vi "UHR-Fleezers Control (host) - 12.6.1.vi"() -> ()   [LabVIEW 2012] (continued)
            n2034 = Bundle("Left"=w2971, "Top"=w2970, "Width"=w2969, "Height"=w2968) -> (w2959:T33)  [unwired: 1 in]
            n2035 = Bundle("Left"=w2967, "Top"=w2966, "Width"=w2965, "Height"=w2964) -> (w2958:T33)  [unwired: 1 in]
            n2036 = Bundle("Left"=w2963, "Top"=w2962, "Width"=w2961, "Height"=w2960) -> (w2957:T33)  [unwired: 1 in]
            n2037 = Build Cluster Array(w2942, w2959, w2958, w2957) -> (w2956:T34)
            n2038 = for {
              tunnel: w2978 -> [w2989]
              tunnel: w2956 -> [w2990] mode=indexing
              shift-right: [w2987] -> w2954
              shift-left: TRUE -> [w2988]
              shift-right: [w2986] -> w2952
              shift-left: _ -> [w2982]
              shift-right: [w2985] -> w2951
              shift-left: _ -> [w2981]
              shift-right: [w2984] -> w2950
              shift-left: _ -> [w2980]
              shift-right: [w2983] -> w2949
              shift-left: _ -> [w2979]
              n2039 = case shown="True" w2988 {
                selector: w2988 -> [w2995 _]
                tunnel: w2990 -> [_ w3004]
                tunnel: w2989 -> [_ w3002]
                tunnel: [w2995 w3000] -> w2987
                tunnel: [w2994 w2999] -> w2986
                tunnel: [w2993 w2998] -> w2985
                tunnel: [w2992 w2997] -> w2984
                tunnel: [w2991 w2996] -> w2983
                tunnel: w2982 -> [w2994 _]
                tunnel: w2981 -> [w2993 _]
                tunnel: w2980 -> [w2992 _]
                tunnel: w2979 -> [w2991 _]
                frame False {
                }
                frame True {
                  n2040 = Unbundle(w3004) -> (w3003:T33)
                  n2041 = call "isclickinwindow.vi"("Image Param"=w3003, "Point32"=w3002) -> ("4 Y"=w2996:i32, "3 Height"=w2997:i32, "2 X"=w2998:i32, "1 Width"=w2999:i32, "In image?"=w3001:bool)  [unwired: 1 in]
                  n2042 = Not(x=w3001) -> (.not. x?=w3000:bool)
                }
              }
            }
            n2043 = Not(x=w2954) -> (.not. x?=w2953:bool)
            n2044 = case shown="True" w2953 {
              tunnel: w2951 -> [_ w3018]
              tunnel: w2949 -> [_ w3017]
              tunnel: w2952 -> [_ w3016]
              tunnel: w2950 -> [_ w3015]
              frame False {
              }
              frame True {
                w3005 = FALSE ("Get Point")
                n2045 = local read "Scan lines (y)"() -> (w3020:u64)
                n2046 = disable-structure shown="Disabled" {
                  frame Disabled {
                  }
                  frame Enabled {
                  }
                }
                n2047 = local read "Actual MCL Inc (V)"() -> (w3014:dbl)
                n2048 = local read "Scan steps (MCL)"() -> (w3019:u64)
                n2049 = Divide "Y Pix/step"(x=w3015, y=w3020) -> (x/y=w3027:dbl)
                n2050 = Divide "Y V/pix"(x=w3014, y=w3027) -> (x/y=w3026:dbl)
                n2051 = Divide "Y half step offset"(x=w3014, y=2.0) -> (x/y=w3028:dbl)
                n2052 = Divide "X pix/step"(x=w3016, y=w3019) -> (x/y=w3025:dbl)
                n2053 = Negate(x=w3028) -> (-x=w3029:dbl)
                n2054 = local read "Initial Y"() -> (w3035:dbl)
                n2055 = Multiply(x=w3017, y=w3026) -> (x*y=w3036:dbl)
                n2056 = Divide "X half step offset"(x=w3014, y=2.0) -> (x/y=w3022:dbl)
                n2057 = Divide "X V/pix"(x=w3014, y=w3025) -> (x/y=w3024:dbl)
                n2058 = Multiply(x=w3014, y=w3019) -> (x*y=w3031:dbl)
                n2059 = Compound Arithmetic op=ADD(w3029, w3036, w3035) -> (w3006:dbl)
                "Pointer Y (V)" <- w3006
                n2060 = Multiply(x=w3024, y=w3018) -> (x*y=w3033:dbl)
                n2061 = Negate(x=w3022) -> (-x=w3021:dbl)
                n2062 = local read "Initial X"() -> (w3034:dbl)
                n2063 = Negate(x=w3033) -> (-x=w3032:dbl)
                n2064 = Compound Arithmetic op=ADD(w3021, w3031, w3034, w3032) -> (w3007:dbl)
                "Pointer X (V)" <- w3007
                n2065 = case shown="True" "Set High F Confocal Spot (X-Y)" {
                  tunnel: w3007 -> [_ w3037]
                  tunnel: w3006 -> [_ w3038]
                  frame False {
                  }
                  frame True {
                    "Confocal Y 2 (V)" <- w3038
                    "Confocal X 2 (V)" <- w3037
                  }
                }
                n2066 = Or(x="Set X Only", y="Set Confocal Spot (X-Y)") -> (x .or. y?=w3010:bool)
                n2067 = Or(x="Set Confocal Spot (X-Y)", y="Set Y Only") -> (x .or. y?=w3009:bool)
                n2068 = case shown="True" w3010 {
                  tunnel: w3007 -> [_ w3039]
                  frame False {
                  }
                  frame True {
                    n2069 = property on="AO2" class="Slide (strict)"("Val(Sgnl)"=w3039) -> ()  [unwired: 2 in, 2 out]
                    "Confocal X 1 (V)" <- w3039
                  }
                }
                n2070 = case shown="True" w3009 {
                  tunnel: w3006 -> [_ w3040]
                  frame False {
                  }
                  frame True {
                    n2071 = property on="AO1" class="Slide (strict)"("Val(Sgnl)"=w3040) -> ()  [unwired: 2 in, 2 out]
                    "Confocal Y 1 (V)" <- w3040
                  }
                }
                n2072 = local write "Set High F Confocal Spot (X-Y)"(w3005) -> ()
                n2073 = local write "Set Confocal Spot (X-Y)"(w3005) -> ()
                n2074 = local write "Set X Only"(w3005) -> ()
                n2075 = local write "Set Y Only"(w3005) -> ()
              }
            }
          }
          frame 3 {
            n2076 = local read "BD 2 Frequency 1 (MHz)"() -> (w3041:dbl)
            n2077 = local read "BD 1 Frequency 1 (MHz)"() -> (w3042:dbl)
            n2078 = local write "Manipulating Trap"(TRUE ("Manipulating Trap")) -> ()
            n2079 = local write "Coords"(T7 {"Horizontal"=0, "Vertical"=0} ("Coords")) -> ()
            n2080 = while {
              tunnel: w3047 -> [w3052]
              tunnel: w3045 -> [w3051]
              tunnel: w3043 -> [w3050]
              tunnel: w3042 -> [w3049]
              tunnel: w3041 -> [w3048]
              stop <- w3053 stop-if-true
              n2081 = event shown="[0] \"Pane\": Mouse Move" {
                selector: _ -> [_ _]
                dyn-events: _ -> [_ _]
                timeout: _ -> [_ _]
                tunnel: ["Force Manip Abort" w3117] -> w3053
                tunnel: w3052 -> [w3060 _]
                tunnel: w3051 -> [w3058 _]
                tunnel: w3050 -> [w3057 _]
                tunnel: w3049 -> [w3056 _]
                tunnel: w3048 -> [w3055 _]
                event Mouse Move {
                  n2082 = event-data() -> ("Time"=w3061:u32, "Coords"=w3062:T7)  [unwired: 3 out]
                  n2083 = Less?(x=w3061, y=w3060) -> (x < y?=w3059:bool)
                  n2084 = case "Makes sure old motion events prior to mouse click aren't used" shown="False" w3059 {
                    tunnel: w3062 -> [w3104 _]
                    tunnel: w3058 -> [w3105 _]
                    tunnel: w3057 -> [w3082 _]
                    tunnel: w3056 -> [w3078 _]
                    tunnel: w3055 -> [w3077 _]
                    frame False {
                      n2085 = Subtract(x=w3104, y=w3105) -> (x-y=w3103:T7)
                      "Coords" <- w3103
                      n2086 = local read "Y RF Frequency Limits (MHz)"() -> (w3063:T16)
                      n2087 = To Double Precision Float(number=w3103) -> (double precision float=w3102:cluster{"Horizontal":dbl, "Vertical":dbl})
                      n2088 = Multiply(x=cluster{"Horizontal":dbl, "Vertical":dbl} {"Horizontal"=-1.0, "Vertical"=1.0}, y="Manipulation Scaling") -> (x*y=w3098:cluster{"Horizontal":dbl, "Vertical":dbl})
                      n2089 = local read "X RF Frequency Limits (MHz)"() -> (w3064:T16)
                      n2090 = Multiply(x=w3102, y=w3098) -> (x*y=w3100:cluster{"Horizontal":dbl, "Vertical":dbl})
                      n2091 = Unbundle By Name(w3100) -> ("Horizontal"=w3095:dbl, "Vertical"=w3099:dbl)
                      n2092 = Unbundle By Name(w3063) -> ("Maximum"=w3066:dbl, "Minimum"=w3065:dbl)
                      n2093 = Boolean To (0,1)(Boolean="Manip. X?") -> (0, 1=w3093:i16)
                      n2094 = Boolean To (0,1)(Boolean="Manip. Y?") -> (0, 1=w3090:i16)
                      n2095 = local read "BD 1 Frequency 2 (MHz)"() -> (w3080:dbl)
                      n2096 = Multiply(x=w3099, y=w3090) -> (x*y=w3092:dbl)
                      n2097 = Multiply(x=w3093, y=w3095) -> (x*y=w3096:dbl)
                      n2098 = local read "BD 2 Frequency 2 (MHz)"() -> (w3079:dbl)
                      n2099 = Unbundle By Name(w3064) -> ("Maximum"=w3068:dbl, "Minimum"=w3067:dbl)
                      n2100 = Add(x=w3077, y=w3092) -> (x+y=w3070:dbl)
                      n2101 = Add(x=w3078, y=w3096) -> (x+y=w3072:dbl)
                      n2102 = In Range and Coerce(upper limit=w3068, x=w3072, lower limit=w3067) -> (coerced(x)=w3071:dbl)  [unwired: 1 out]
                      n2103 = In Range and Coerce(upper limit=w3066, x=w3070, lower limit=w3065) -> (coerced(x)=w3069:dbl)  [unwired: 1 out]
                      n2104 = Subtract(x=w3071, y=w3080) -> (x-y=w3089:dbl)
                      n2105 = Subtract(x=w3069, y=w3079) -> (x-y=w3088:dbl)
                      n2106 = Square(x=w3089) -> (x^2=w3087:dbl)
                      n2107 = Square(x=w3088) -> (x^2=w3086:dbl)
                      n2108 = Add(x=w3087, y=w3086) -> (x+y=w3085:dbl)
                      n2109 = Square Root(x=w3085) -> (sqrt(x)=w3081:dbl)
                      n2110 = In Range and Coerce(upper limit="Limit Max (MHz)", x=w3081, lower limit="Limit Min (MHz)") -> (In Range?=w3074:bool)  [unwired: 1 out]
                      n2111 = Not(x="Limits Enable") -> (.not. x?=w3073:bool)
                      n2112 = Or(x=w3074, y=w3073) -> (x .or. y?=w3075:bool)
                      n2113 = case shown="True" w3075 {
                        tunnel: w3082 -> [_ w3115]
                        tunnel: w3081 -> [_ w3106]
                        tunnel: w3071 -> [_ w3113]
                        tunnel: w3080 -> [_ w3112]
                        tunnel: w3069 -> [_ w3111]
                        tunnel: w3079 -> [_ w3110]
                        tunnel: w3064 -> [_ w3108]
                        tunnel: w3063 -> [_ w3107]
                        frame False {
                        }
                        frame True {
                          n2114 = local read "BD 1 Frequency 3 (MHz)"() -> (w3114:dbl)
                          n2115 = local read "BD 2 Frequency 3 (MHz)"() -> (w3109:dbl)
                          n2116 = local write "Trap Delta (MHz)"(w3106) -> ()
                          n2117 = call "set RF board frequency - interlace.vi"("Board 2 Frequency Limits"=w3107, "Board 1 Frequency Limits"=w3108, "FPGA VI Reference In"=w3115, "Board 2 Frequency 3 (MHz)"=w3109, "Board 1 Frequency 3 (MHz)"=w3114, "Board 2 Frequency 2 (MHz)"=w3110, "Board 2 Frequency 1 (MHz)"=w3111, "Board 1 Frequency 2 (MHz)"=w3112, "Board 1 Frequency 1  (MHz)"=w3113) -> ()  [unwired: 1 in, 2 out]
                          n2118 = local write "BD 2 Frequency 1 (MHz)"(w3111) -> ()
                          n2119 = local write "BD 1 Frequency 1 (MHz)"(w3113) -> ()
                        }
                      }
                    }
                    frame True {
                    }
                  }
                }
                event Mouse Up {
                  n2120 = event-data() -> ("Button"=w3116:u16)  [unwired: 8 out]
                  n2121 = case shown="3" w3116 {
                    tunnel: [FALSE TRUE] -> w3117
                    frame 0, Default {
                    }
                    frame 3 {
                      n2122 = local read "Trap Delta (MHz)"() -> (w3119:dbl)
                      n2123 = property on="Initial delta (MHz)" class="DigNum (strict)"("Val(Sgnl)"=w3119) -> ()  [unwired: 2 in, 2 out]
                      n2124 = local write "Manipulating Trap"(FALSE ("Manipulating Trap")) -> ()
                    }
                  }
                }
              }
            }
          }
        }
      }
      event Mouse Move {
        n2125 = event-data() -> ()  [unwired: 6 out]
      }
    }
    n2126 = local read "Stop All"() -> (w2935:bool)
    n2127 = node-c288() -> ()  [unwired: 2 out]
  }
  n2128 = timed-loop "Main data acquisition loop (get data, process data for display, and save data to disk)" {
    tunnel: w16 -> [w3431]
    tunnel: w88 -> [w3430]
    tunnel: [w3460] -> w292
    tunnel: [w3455] -> w290
    timing: w200 -> [_]
    timing-out: [_] -> w199
    tunnel: w105 -> [w3284]
    stop <- "Stop All" stop-if-true
    w3201 = "Initialize"
    # "Fluorescence data into FIFO for external control vi's\n(e.g., fluorescence triggering) - Duncan Nall"
    n2129 = node-c288() -> ()  [unwired: 2 out]
    n2130 = First Call?() -> (First Call?: T/F=w3236:bool)
    n2131 = Or(x="Reset", y=w3236) -> (x .or. y?=w3237:bool)
    n2132 = local read "Flushing P1"() -> (w3156:bool)
    n2133 = case "Reset data stream (manual reset or at begining of some rastering and imaging)" shown="True" w3237 {
      tunnel: w3431 -> [w4502 w4510]
      tunnel: w3430 -> [w4501 w4509]
      tunnel: [w4502 w4504] -> w3426
      tunnel: [w4501 w4503] -> w3425
      frame False {
      }
      frame True {
        w4507 = TRUE ("AI to FIFO")
        n2134 = local write "Overflow (data lost)"(FALSE ("Overflow (data lost)")) -> ()
        n2135 = call "reset FPGA DMA.vi"("error in"=w4509, "FPGA VI Reference In"=w4510) -> ("error out"=w4505:errorcluster, "FPGA VI Reference Out"=w4506:T20)
        n2136 = xnode "Read/Write Control"("FPGA VI Reference In"=w4506, "error in"=w4505, "AI to FIFO"=w4507, "APD to FIFO"=w4507) -> ("FPGA VI Reference Out"=w4504:T20, "error out"=w4503:errorcluster)
      }
    }
    n2137 = case shown="True" w3156 {
      frame False {
      }
      frame True {
        n2138 = local read "Flush rate (uL/m) P1"() -> (w3490:dbl)
        n2139 = local read "HP1 Flush Time (s)"() -> (w3499:dbl)
        n2140 = local read "DMA Update Period (s)"() -> (w3493:dbl)
        n2141 = Divide(x=w3490, y=60.0) -> (x/y=w3491:dbl)
        n2142 = Divide(x=w3499, y=w3493) -> (x/y=w3488:dbl)
        n2143 = feedback #1(0) -> (w3497:i32)
        n2144 = Increment(x=w3497) -> (x+1=w3487:i32)
        n2145 = Greater?(x=w3487, y=w3488) -> (0:w3496:bool)
        n2146 = Compound Arithmetic op=MULTIPLY(w3493, w3487, w3491) -> (→"P1 Flush Volume (uL)":dbl)
        n2147 = Divide(x=w3487, y=w3488) -> (x/y=→"P1 Flushing Bar":dbl)
        n2148 = case shown="True" w3496 {
          tunnel: w3487 -> [w3500 _]
          tunnel: [w3500 0] -> w3495
          frame False {
          }
          frame True {
            w3501 = FALSE ("Flushing P1")
            n2149 = local write "Inject Pump 1"(w3501) -> ()
            n2150 = local write "Flushing P1"(w3501) -> ()
            n2151 = property on="Clear Volume P1" class="Bool (strict)"("Val(Sgnl)"=TRUE ("Value (Signaling)")) -> ()  [unwired: 2 in, 2 out]
          }
        }
        n2152 = feedback-in #1(w3495) -> ()
      }
    }
    n2153 = Or(x="Start AOD Scan", y="Trap Raster Scan") -> (x .or. y?=w3382:bool)
    n2154 = case "Start AOM raster scan" shown="True" w3382 {
      tunnel: w3426 -> [w4352 w4362]
      tunnel: w3425 -> [w4351 w4361]
      tunnel: [w4352 w4355] -> w3424
      tunnel: [w4351 w4354] -> w3423
      frame False {
      }
      frame True {
        n2155 = case shown="True" "Restart DMA? (AOD)" {
          tunnel: [w4400 w4402] -> w4356
          tunnel: [w4399 w4401] -> w4357
          tunnel: w4362 -> [w4400 w4404]
          tunnel: w4361 -> [w4399 w4403]
          frame False {
          }
          frame True {
            n2156 = local write "Overflow (data lost)"(FALSE ("Overflow (data lost)")) -> ()
            n2157 = call "reset FPGA DMA.vi"("error in"=w4403, "FPGA VI Reference In"=w4404) -> ("error out"=w4401:errorcluster, "FPGA VI Reference Out"=w4402:T20)
          }
        }
        n2158 = local write "Trap Raster Scan"(FALSE ("Trap Raster Scan")) -> ()
        n2159 = case shown="True" "Move MCL Also?" {
          tunnel: w4357 -> [w4365 w4394]
          tunnel: w4356 -> [w4366 w4395]
          tunnel: [w4364 w4398] -> w4355
          tunnel: [w4363 w4397] -> w4354
          frame False {
            w4367 = TRUE ("AI to FIFO")
            n2160 = xnode "Read/Write Control"("FPGA VI Reference In"=w4366, "error in"=w4365, "AI to FIFO"=w4367, "APD to FIFO"=w4367, "Start scan"=w4367) -> ("FPGA VI Reference Out"=w4364:T20, "error out"=w4363:errorcluster)
          }
          frame True {
            w4391 = FALSE ("1D or 2D Scan?")
            w4396 = TRUE ("AI to FIFO")
            # "Count for MCL loop"
            # "N total cycles"
            # "N steps"
            # "V_int"
            n2161 = local read "Scan Range (nm)"() -> (w4373:dbl)
            n2162 = local read "Number of F/B Scans (AOD)"() -> (w4390:u16)
            n2163 = Sign(1:w4373) -> (0:w4372:dbl)
            n2164 = Compound Arithmetic op=MULTIPLY(w4373, "MCL Step Position Ratio", "MCL/AOM Scale Tweak") -> (w4377:dbl)
            n2165 = Negate(x=w4372) -> (-x=w4369:dbl)
            n2166 = Multiply(x=w4369, y="MCL Step Increment (V_int)") -> (x*y=w4371:dbl)
            n2167 = Divide(x=w4377, y="MCL X Cal (nm/V)") -> (x/y=w4383:dbl)
            n2168 = Multiply(x=32767.0 ("y"), y=w4383) -> (x*y=w4389:dbl)
            n2169 = local read "Total Counts (ticks)"() -> (w4374:u16)
            n2170 = local read "Cycles/step (AOD)"() -> (w4385:u64)
            n2171 = local read "Scan steps (AOD)"() -> (w4386:u64)
            n2172 = Divide(x=w4389, y=10.0) -> (x/y=w4382:dbl)
            n2173 = Divide(x=w4382, y="MCL Step Increment (V_int)") -> (x/y=w4380:dbl)
            n2174 = Absolute Value(x=w4380) -> (abs(x)=w4368:dbl)
            n2175 = Compound Arithmetic op=MULTIPLY(w4386, w4385, w4374) -> (w4381:u64)
            n2176 = local write "wait to reset values"(w4396) -> ()
            n2177 = local write "MCL Scanning"(w4396) -> ()
            n2178 = Divide(x=w4381, y=w4368) -> (x/y=w4378:dbl)
            "MCL Count" <- w4378
            n2179 = xnode "Read/Write Control"("FPGA VI Reference In"=w4395, "error in"=w4394, "Scan steps (MCL)"=w4368, "Number of scans (MCL)"=w4390, "Cycles per step (MCL)"=u64 1, "Scan freq.  increment (MCL)"=w4371, "1D or 2D Scan?"=w4391, "MCL Scan Axis"=w4391, "Cont. Scan (MCL)"=w4391, "MCL count"=w4378) -> ("FPGA VI Reference Out"=w4393:T20, "error out"=w4392:errorcluster)
            n2180 = xnode "Read/Write Control"("FPGA VI Reference In"=w4393, "error in"=w4392, "AI to FIFO"=w4396, "APD to FIFO"=w4396, "Start scan"=w4396, "Start scan (MCL)"=w4396) -> ("FPGA VI Reference Out"=w4398:T20, "error out"=w4397:errorcluster)
          }
        }
        "Raster Scanning..." <- TRUE ("Scanning...")
      }
    }
    n2181 = local read "Flushing P3"() -> (w3157:bool)
    n2182 = case "Keep track of when Harvard Pump 3 is done flushing" shown="True" w3157 {
      frame False {
      }
      frame True {
        n2183 = local read "Flush rate (uL/m) P3"() -> (w3507:dbl)
        n2184 = local read "DMA Update Period (s)"() -> (w3509:dbl)
        n2185 = local read "HP3 Flush Time (s)"() -> (w3516:dbl)
        n2186 = Divide(x=w3507, y=60.0) -> (x/y=w3505:dbl)
        n2187 = feedback #2(0) -> (w3514:i32)
        n2188 = Increment(x=w3514) -> (x+1=w3508:i32)
        n2189 = Divide(x=w3516, y=w3509) -> (x/y=w3510:dbl)
        n2190 = Greater?(x=w3508, y=w3510) -> (0:w3513:bool)
        n2191 = Compound Arithmetic op=MULTIPLY(w3509, w3508, w3505) -> (→"P3 Flush Volume (uL)":dbl)
        n2192 = case shown="True" w3513 {
          tunnel: w3508 -> [w3517 _]
          tunnel: [w3517 0] -> w3512
          frame False {
          }
          frame True {
            w3518 = FALSE ("Flushing P3")
            n2193 = local write "Inject Pump 3"(w3518) -> ()
            n2194 = local write "Flushing P3"(w3518) -> ()
            n2195 = property on="Clear Volume P3" class="Bool (strict)"("Val(Sgnl)"=TRUE ("Value (Signaling)")) -> ()  [unwired: 2 in, 2 out]
          }
        }
        n2196 = feedback-in #2(w3512) -> ()
        n2197 = Divide(x=w3508, y=w3510) -> (x/y=→"P3 Flushing Bar":dbl)
      }
    }
    n2198 = And(x="Save scans", y=w3382) -> (x .and. y?=w3422:bool)
    n2199 = Compound Arithmetic op=OR("Start MCL Scan", "Confocal Image", "Confocal Linescan") -> (w3380:bool)
    n2200 = And(x="Save Data (MCL)", y=w3380) -> (x .and. y?=w3421:bool)
    n2201 = case "Start MCL raster scan" shown="True" w3380 {
      tunnel: w3424 -> [w3964 w3980]
      tunnel: w3423 -> [w3963 w3979]
      tunnel: [w3964 w3975] -> w3283
      tunnel: [w3963 w3974] -> w3282
      tunnel: [FALSE w3973] -> w3407
      tunnel: "Start MCL Scan" -> [_ w3968]
      tunnel: "Confocal Image" -> [_ w3967]
      tunnel: "Confocal Linescan" -> [_ _]
      frame False {
      }
      frame True {
        w3973 = TRUE
        n2202 = case shown="True" "Restart DMA? (MCL)" {
          tunnel: [w4025 w4027] -> w3978
          tunnel: [w4024 w4026] -> w3977
          tunnel: w3980 -> [w4025 w4030]
          tunnel: w3979 -> [w4024 w4029]
          frame False {
          }
          frame True {
            n2203 = call "reset FPGA DMA.vi"("error in"=w4029, "FPGA VI Reference In"=w4030) -> ("error out"=w4026:errorcluster, "FPGA VI Reference Out"=w4027:T20)
            n2204 = local write "Overflow (data lost)"(FALSE ("Overflow (data lost)")) -> ()
          }
        }
        n2205 = case shown="False" w3968 {
          selector: w3968 -> [_ w3984]
          tunnel: w3967 -> [w3983 _]
          tunnel: [w3983 w3984] -> w3966
          frame False {
            n2206 = property on="2D or 1D Scan" class="Bool (strict)"("Val(Sgnl)"=w3983) -> ()  [unwired: 2 in, 2 out]
            n2207 = property on="Confocal Image" class="Bool (strict)"("Value"=FALSE ("Start Confocal Map")) -> ()  [unwired: 2 in, 2 out]
          }
          frame True {
          }
        }
        n2208 = local write "MCL Scanning"(w3973) -> ()
        n2209 = local read "AO1"() -> (w3970:dbl)
        n2210 = local read "AO2"() -> (w3969:dbl)
        n2211 = case shown="True" "Center Scan" {
          tunnel: w3978 -> [w3991 w4023]
          tunnel: w3977 -> [w3990 w4022]
          tunnel: [w3989 w4021] -> w3975
          tunnel: [w3988 w4020] -> w3974
          tunnel: [w3986 w4007] -> w3972
          tunnel: [w3985 w4006] -> w3971
          tunnel: w3970 -> [w3986 w4012]
          tunnel: w3969 -> [w3985 w4015]
          tunnel: w3966 -> [_ _]
          frame False {
            w3987 = TRUE ("AI to FIFO")
            n2212 = xnode "Read/Write Control"("FPGA VI Reference In"=w3991, "error in"=w3990, "AI to FIFO"=w3987, "APD to FIFO"=w3987, "Start scan (MCL)"=w3987) -> ("FPGA VI Reference Out"=w3989:T20, "error out"=w3988:errorcluster)
          }
          frame True {
            w4019 = TRUE ("AI to FIFO")
            n2213 = local read "Scan steps (MCL)"() -> (w3998:u64)
            n2214 = local read "Scan lines (y)"() -> (w3994:u64)
            n2215 = local read "Fast Scan Dir"() -> (w4005:bool)
            n2216 = local read "Actual MCL Inc (V)"() -> (w3995:dbl)
            n2217 = Decrement(x=w3994) -> (x-1=w3993:u64)
            n2218 = Decrement(x=w3998) -> (x-1=w3997:u64)
            n2219 = Multiply(x=w3995, y=w3993) -> (x*y=w3992:dbl)
            n2220 = Divide(x=w3992, y=2.0) -> (x/y=w4002:dbl)
            n2221 = Multiply(x=w3995, y=w3997) -> (x*y=w3996:dbl)
            n2222 = Divide(x=w3996, y=2.0) -> (x/y=w4001:dbl)
            n2223 = Select(t=w4001, s=w4005, f=w4002) -> (s? t:f=w4000:dbl)
            n2224 = Select(t=w4002, s=w4005, f=w4001) -> (s? t:f=w4004:dbl)
            n2225 = Subtract(x=w4012, y=w4004) -> (x-y=w4003:dbl)
            n2226 = Subtract(x=w4015, y=w4000) -> (x-y=w3999:dbl)
            n2227 = local read "2D or 1D Scan"() -> (w4017:bool)
            n2228 = Not(x=w4005) -> (.not. x?=w4011:bool)
            n2229 = Not(x=w4017) -> (.not. x?=w4013:bool)
            n2230 = And(x=w4005, y=w4013) -> (x .and. y?=w4014:bool)
            n2231 = And(x=w4013, y=w4011) -> (x .and. y?=w4016:bool)
            n2232 = Select(t=w4015, s=w4016, f=w3999) -> (s? t:f=w4006:dbl)
            n2233 = Select(t=w4012, s=w4014, f=w4003) -> (s? t:f=w4007:dbl)
            n2234 = call "Volt to I16.vi"("Voltage In"=w4007) -> ("I16 Voltage Out"=w4010:i16)
            n2235 = call "Volt to I16.vi"("Voltage In"=w4006) -> ("I16 Voltage Out"=w4009:i16)
            n2236 = xnode "Read/Write Control"("FPGA VI Reference In"=w4023, "error in"=w4022, "AI to FIFO"=w4019, "APD to FIFO"=w4019, "Start scan (MCL)"=w4019, "AO1"=w4010, "AO2"=w4009) -> ("FPGA VI Reference Out"=w4021:T20, "error out"=w4020:errorcluster)
          }
        }
        "Initial Y" <- w3972
        "Initial X" <- w3971
        n2237 = local write "Tab Control 6"(T3."Imaging" ("Tab Control 6")) -> ()
        "wait to reset values" <- w3973
      }
    }
    n2238 = local read "APD Elements/DMA read"() -> (w3127:u32)
    n2239 = local read "Trap AI Elements/DMA read"() -> (w3345:u32)
    n2240 = xnode "Get APD Data"("FPGA VI Reference In"=w3283, "error in"=w3282, "Number of Elements"=w3127, "Timeout (ms)"=-1) -> ("Data"=w3314:u32[], "Elements Remaining"=→"APD FIFO Elements Remaining":u32)  [unwired: 2 out]
    n2241 = local read "Trap Pos Elements/DMA read"() -> (w3279:u32)
    n2242 = xnode "Invoke Method"("FPGA VI Reference In"=w3283, "error in"=w3282, "Number of Elements"=w3279, "Timeout (ms)"=-1) -> ("Data"=w3243:u16[], "Elements Remaining"=→"Trap Pos FIFO El Remaining":u32)  [unwired: 2 out]
    n2243 = xnode "Get Trap Data"("FPGA VI Reference In"=w3283, "error in"=w3282, "Number of Elements"=w3345, "Timeout (ms)"=-1 ("Timeout")) -> ("FPGA VI Reference Out"=w3178:T20, "error out"=w3177:errorcluster, "Data"=w3244:i16[], "Elements Remaining"=w3468:u32)
    "FIFO El. Rem." <- w3468
    n2244 = local read "DMA Update Period (s)"() -> (w3346:dbl)
    n2245 = local read "Trap AI FIFO Depth"() -> (w3470:u32)
    n2246 = local read "Number of APDs"() -> (w3146:u8)
    n2247 = Decimate 1D Array(w3243) -> (w3240:u16[], w3242:u16[], w3241:u16[])
    n2248 = feedback #3(0.0) -> (w3272:dbl)
    n2249 = Add(x=w3346, y=w3272) -> (x+y=w3444:dbl)
    n2250 = feedback-in #3(w3444) -> ()
    n2251 = To Time Stamp(1:w3272) -> (0:w3271:timestamp)
    n2252 = Subtract(x=w3470, y=w3345) -> (x-y=w3469:u32)
    n2253 = To Unsigned Long Integer(number=w3240) -> (unsigned 32bit integer=w3239:u32[])
    n2254 = Join Numbers(hi=w3242, lo=w3241) -> ((hi.lo)=w3238:u32[])
    n2255 = Divide(x=w3468, y=w3469) -> (x/y=w3467:dbl)
    "Buffer Status" <- w3467
    n2256 = case "Deinterlace APD signals" shown="3, Default" w3146 {
      tunnel: [w3480 w3486] -> w3126
      tunnel: w3314 -> [w3481 w3485]
      tunnel: [w3479 w3484] -> w3125
      tunnel: [w3478 w3482] -> w3123
      frame 3, Default {
        n2257 = Decimate 1D Array "APD signals"(w3481) -> (w3480:u32[], w3479:u32[], w3478:u32[])
      }
      frame 2 {
        n2258 = Decimate 1D Array "APD signals"(w3485) -> (w3486:u32[], w3484:u32[])
        n2259 = Multiply(x=w3484, y=u32 0) -> (x*y=w3482:u32[])
      }
    }
    n2260 = Join Numbers(hi=w3239, lo=w3238) -> ((hi.lo)=w3232:u64[])
    n2261 = call "IR AOM word to freq - vec.vi"("Frequency Word In (double vec)"=w3232) -> ("Frequency Out"=w3278:dbl[])
    n2262 = Equal?(x=w3467, y=1.0) -> (x = y?=w3465:bool)
    n2263 = case "Alert buffer overflow" shown="True" w3465 {
      frame False {
      }
      frame True {
        n2264 = call <vilib>:"Beep.vi"() -> ()  [unwired: 3 in, 9 out]
        "Overflow (data lost)" <- TRUE ("Overflow (data lost)")
      }
    }
    n2265 = Decimate 1D Array(w3278) -> (w3277:dbl[], w3276:dbl[])
    n2266 = Build Array(w3277, w3276) -> (w3275:dbl[][])
    n2267 = Bundle(w3126, w3125, w3123) -> (w3130:cluster{u32[], u32[], u32[]})  [unwired: 1 in]
    n2268 = Build Array(w3126, w3125, w3123) -> (w3404:u32[][])
    n2269 = for {
      tunnel: w3126 -> [w3476] mode=indexing
      n2270 = call "Smart Buffer (DBL) 1.vi"("new element [write]"=w3476, "mode"=T21."write") -> ()  [unwired: 4 in, 6 out]
    }
    n2271 = local read "APD Integration Time (s)"() -> (w3141:dbl)
    n2272 = To Double Precision Float(number=w3404) -> (double precision float=w3405:dbl[][])
    n2273 = feedback #4 "APD3"(w3123) -> (w3124:u32[])
    n2274 = feedback #5 "APD2"(w3125) -> (w3301:u32[])
    n2275 = feedback #6 "APD1"(w3126) -> (w3403:u32[])
    n2276 = Build Array (concatenate)(w3301, w3125) -> (w3300:u32[])
    n2277 = Build Array (concatenate)(w3124, w3123) -> (w3122:u32[])
    n2278 = Build Array (concatenate)(w3403, w3126) -> (w3400:u32[])
    n2279 = for {
      tunnel: w3125 -> [w3475] mode=indexing
      n2280 = call "Smart Buffer (DBL) 2.vi"("new element [write]"=w3475, "mode"=T21."write") -> ()  [unwired: 4 in, 6 out]
    }
    n2281 = Array Size(array=w3400) -> (size(s)=w3397:i32)
    n2282 = Array Size(array=w3126) -> (size(s)=w3399:i32)
    n2283 = Multiply(x=w3399, y="APD Ave N") -> (x*y=w3398:dbl)
    n2284 = Greater?(x=w3397, y=w3398) -> (0:w3401:bool)
    n2285 = Bundle("APD 1", "APD 2", "APD 3") -> (w3437:cluster{string, string, string})  [unwired: 1 out]
    n2286 = local read "Trap Sets"() -> (w3344:u32)
    n2287 = case shown="True" w3401 {
      tunnel: w3400 -> [w3779 w3788]
      tunnel: [w3779 w3786] -> w3351
      tunnel: w3398 -> [_ w3781]
      tunnel: w3397 -> [_ w3787]
      tunnel: w3300 -> [w3778 w3785]
      tunnel: [w3778 w3784] -> w3298
      tunnel: w3122 -> [w3777 w3783]
      tunnel: [w3777 w3780] -> w3142
      frame False {
      }
      frame True {
        n2288 = Subtract(x=w3787, y=w3781) -> (x-y=w3782:dbl)
        n2289 = Array Subset "APD3"(array=w3783, index=w3782, length=w3781) -> (w3780:u32[])
        n2290 = Array Subset "APD2"(array=w3785, index=w3782, length=w3781) -> (w3784:u32[])
        n2291 = Array Subset "APD1"(array=w3788, index=w3782, length=w3781) -> (w3786:u32[])
      }
    }
    n2292 = feedback-in #4(w3142) -> ()
    n2293 = feedback-in #5(w3298) -> ()
    n2294 = feedback-in #6(w3351) -> ()
    n2295 = Cluster To Array(cluster=w3437) -> (array=w3434:string[])
    n2296 = for "APD" {
      tunnel: w3405 -> [w4035] mode=indexing
      tunnel: w3141 -> [w4042]
      tunnel: [w4038] -> w3302 mode=indexing
      tunnel: "APD Disp. Scale" -> [w4039]
      tunnel: w3434 -> [w4037] mode=indexing
      tunnel: "APD Disp. Downsample" -> [w4033]
      tunnel: [w4036] -> w3433
      workers-P: _ -> [_]
      tunnel: w3271 -> [w4032]
      n2297 = call "integrate 1D array interval - double.vi"("Ave N"=w4033, "Array In"=w4035) -> ("Array Out"=w4034:dbl[])  [unwired: 1 out]
      n2298 = Multiply(x=w4042, y=w4033) -> (x*y=w4036:dbl)
      n2299 = Divide(x=w4034, y=w4039) -> (x/y=w4040:dbl[])
      n2300 = Bundle By Name("t0"=w4032, "Y"=w4040, "dt"=w4036) -> (w4041:waveform(dbl))  [unwired: 1 out]
      n2301 = Set Waveform Attribute(5:w4037, 6:"NI_ChannelName" ("name"), 7:w4041) -> (3:w4038:waveform(dbl))  [unwired: 1 in, 2 out]
    }
    "APD Display Period (s)" <- w3433
    n2302 = Reciprocal(x=w3433) -> (1/x=→"APD Display Freq. (Hz)":dbl)
    n2303 = case "Deinterlace trap data, average down PSD" shown="2" w3344 {
      tunnel: w3244 -> [w4060 w4125]
      tunnel: [w4057 w4122] -> w3337
      tunnel: [w4060 w4124] -> w3235
      tunnel: "Detector Type" -> [w4059 w4120]
      tunnel: [w4058 w4123] -> w3336
      tunnel: [w4056 w4121] -> w3442
      frame 1, Default {
        n2304 = Divide(x=w4060, y=3276.7) -> (x/y=w4061:dbl[])
        n2305 = Decimate 1D Array(w4061) -> (w4070:dbl[], w4069:dbl[], w4068:dbl[], w4067:dbl[], w4066:dbl[], w4065:dbl[], w4064:dbl[], w4063:dbl[])
        n2306 = case shown="\"IR-QPD + PSD + FB-QPD position\"" w4059 {
          tunnel: w4070 -> [w4094 w4119]
          tunnel: w4069 -> [w4093 w4118]
          tunnel: w4068 -> [w4078 w4096]
          tunnel: w4067 -> [w4079 w4106]
          tunnel: w4066 -> [w4092 w4117]
          tunnel: w4065 -> [w4091 w4116]
          tunnel: w4064 -> [w4075 w4097]
          tunnel: w4063 -> [w4074 w4095]
          tunnel: [w4073 w4103] -> w4058
          tunnel: [w4072 w4102] -> w4057
          tunnel: [w4071 w4101] -> w4056
          frame "IR-QPD + PSD + FB-QPD", Default {
            w4071 = 0  # Channel pattern
            n2307 = Divide(x=w4094, y=w4079) -> (x/y=w4081:dbl[])
            n2308 = Divide(x=w4093, y=w4079) -> (x/y=w4080:dbl[])
            n2309 = Divide(x=w4092, y=w4075) -> (x/y=w4077:dbl[])
            n2310 = Divide(x=w4091, y=w4074) -> (x/y=w4076:dbl[])
            n2311 = Build Array(w4081, w4080, w4079, w4078, w4077, w4076, w4075, w4074) -> (w4072:dbl[][])
            n2312 = Bundle("T1 Y", "T1 X", "T1 Sum", "FB Sum", "PSD Y", "PSD X", "PSD Y Sum", "PSD X Sum") -> (w4090:T41)  [unwired: 1 out]
            n2313 = Cluster To Array(cluster=w4090) -> (array=w4073:string[])
          }
          frame "IR-QPD + PSD + FB-QPD position" {
            w4101 = 3  # Channel pattern
            n2314 = Negate(x=w4097) -> (-x=w4098:dbl[])
            n2315 = Divide(x=w4119, y=w4106) -> (x/y=w4108:dbl[])
            n2316 = Divide(x=w4118, y=w4106) -> (x/y=w4107:dbl[])
            n2317 = Divide(x=w4117, y=w4097) -> (x/y=w4105:dbl[])
            n2318 = Divide(x=w4116, y=w4098) -> (x/y=w4104:dbl[])
            n2319 = Build Array(w4108, w4107, w4106, w4095, w4096, w4105, w4104, w4097) -> (w4102:dbl[][])
            n2320 = Bundle("T1 Y", "T1 X", "T1 Sum", "FB X", "FB Sum", "PSD Y", "PSD X", "PSD Y Sum") -> (w4115:T41)  [unwired: 1 out]
            n2321 = Cluster To Array(cluster=w4115) -> (array=w4103:string[])
          }
        }
      }
      frame 2 {
        n2322 = case shown="\"IR-QPD + PSD + FB-QPD X position\"" w4120 {
          tunnel: w4125 -> [w4187 w4259 w4330]
          tunnel: [w4126 w4250 w4261] -> w4124
          tunnel: [w4153 w4241 w4308] -> w4123
          tunnel: [w4152 w4204 w4275] -> w4122
          tunnel: [w4146 w4239 w4306] -> w4121
          frame "IR-QPD + PSD + FB-QPD", Default {
            w4146 = 1  # Channel pattern
            # "time average x2 the 4th signal and the 4 psd signals (detection laser)"
            # "deinterlace 3 signals from qpd"
            n2323 = Decimate 1D Array(w4187) -> (w4186:i16[], w4185:i16[], w4151:i16[], w4184:i16[], w4174:i16[], w4172:i16[], w4171:i16[], w4169:i16[])
            n2324 = Decimate 1D Array(w4151) -> (w4150:i16[], w4149:i16[])
            n2325 = Decimate 1D Array(w4186) -> (w4183:i16[], w4155:i16[])
            n2326 = Decimate 1D Array(w4185) -> (w4182:i16[], w4180:i16[])
            n2327 = Decimate 1D Array(w4184) -> (w4181:i16[], w4179:i16[])
            n2328 = call "downsample 1D array - double.vi"("Ave N"=2.0, "Array In"=w4174) -> ("Array Out"=w4173:dbl[])  [unwired: 1 out]
            n2329 = call "downsample 1D array - double.vi"("Ave N"=2.0, "Array In"=w4172) -> ("Array Out"=w4154:dbl[])  [unwired: 1 out]
            n2330 = call "downsample 1D array - double.vi"("Ave N"=2.0, "Array In"=w4171) -> ("Array Out"=w4170:dbl[])  [unwired: 1 out]
            n2331 = call "downsample 1D array - double.vi"("Ave N"=2.0, "Array In"=w4169) -> ("Array Out"=w4168:dbl[])  [unwired: 1 out]
            n2332 = Interleave 1D Arrays(w4183, w4182, w4181, w4155, w4180, w4179, w4150, w4149, w4173, w4154, w4170, w4168) -> (w4167:dbl[])
            n2333 = Divide(x=w4167, y=3276.7) -> (x/y=w4166:dbl[])
            n2334 = Decimate 1D Array(w4166) -> (w4165:dbl[], w4164:dbl[], w4163:dbl[], w4162:dbl[], w4161:dbl[], w4160:dbl[], w4148:dbl[], w4147:dbl[], w4159:dbl[], w4158:dbl[], w4157:dbl[], w4156:dbl[])
            n2335 = Divide(x=w4165, y=w4163) -> (x/y=w4133:dbl[])
            n2336 = Divide(x=w4164, y=w4163) -> (x/y=w4132:dbl[])
            n2337 = Divide(x=w4162, y=w4160) -> (x/y=w4131:dbl[])
            n2338 = Divide(x=w4161, y=w4160) -> (x/y=w4130:dbl[])
            n2339 = Divide(x=w4159, y=w4157) -> (x/y=w4129:dbl[])
            n2340 = Divide(x=w4158, y=w4156) -> (x/y=w4128:dbl[])
            n2341 = Build Array(w4133, w4132, w4163, w4131, w4130, w4160, w4148, w4147, w4129, w4128, w4157, w4156) -> (w4152:dbl[][])
            n2342 = Bundle("T1 Y", "T1 X", "T1 Sum", "T2 Y", "T2 X", "T2 Sum", "T1 FB Sum", "T2 FB Sum", "PSD Y", "PSD X", "PSD Y Sum", "PSD X Sum") -> (w4134:T42)  [unwired: 1 out]
            n2343 = To Word Integer(number=w4167) -> (16bit integer=w4126:i16[])
            n2344 = Cluster To Array(cluster=w4134) -> (array=w4153:string[])
          }
          frame "IR-QPD + PSD + FB-QPD X position" {
            w4239 = 2  # Channel pattern
            # "time average x2 the 3 psd signals (detection laser)"
            # "deinterlace 3 signals from qpds"
            n2345 = Decimate 1D Array(w4259) -> (w4258:i16[], w4257:i16[], w4240:i16[], w4256:i16[], w4202:i16[], w4199:i16[], w4196:i16[], w4227:i16[])
            n2346 = Select(t=i16 -1, s="Flip X Sign", f=i16 1) -> (s? t:f=w4192:i16)
            n2347 = Multiply(x=w4257, y=w4192) -> (x*y=w4193:i16[])
            n2348 = Decimate 1D Array(w4240) -> (w4225:i16[], w4223:i16[])
            n2349 = Decimate 1D Array(w4258) -> (w4255:i16[], w4242:i16[])
            n2350 = Decimate 1D Array(w4193) -> (w4254:i16[], w4252:i16[])
            n2351 = Decimate 1D Array(w4256) -> (w4253:i16[], w4251:i16[])
            n2352 = Decimate 1D Array(w4227) -> (w4226:i16[], w4224:i16[])
            n2353 = call "downsample 1D array - I16.vi"("Ave N"=2.0, "Array In"=w4202) -> ("Array Out"=w4200:i16[])  [unwired: 1 in]
            n2354 = call "downsample 1D array - I16.vi"("Ave N"=2.0, "Array In"=w4196) -> ("Array Out"=w4194:i16[])  [unwired: 1 in]
            n2355 = call "downsample 1D array - I16.vi"("Ave N"=2.0, "Array In"=w4199) -> ("Array Out"=w4197:i16[])  [unwired: 1 in]
            n2356 = Interleave 1D Arrays(w4255, w4254, w4253, w4242, w4252, w4251, w4226, w4225, w4224, w4223, w4200, w4197, w4194) -> (w4250:i16[])
            n2357 = Divide(x=w4250, y=3276.7) -> (x/y=w4249:dbl[])
            n2358 = Decimate 1D Array(w4249) -> (w4248:dbl[], w4247:dbl[], w4246:dbl[], w4245:dbl[], w4244:dbl[], w4243:dbl[], w4215:dbl[], w4213:dbl[], w4212:dbl[], w4210:dbl[], w4209:dbl[], w4208:dbl[], w4205:dbl[])
            n2359 = Negate(x=w4205) -> (-x=w4203:dbl[])
            n2360 = Divide(x=w4209, y=w4205) -> (x/y=w4207:dbl[])
            n2361 = Divide(x=w4208, y=w4203) -> (x/y=w4206:dbl[])
            n2362 = Divide(x=w4248, y=w4246) -> (x/y=w4231:dbl[])
            n2363 = Divide(x=w4247, y=w4246) -> (x/y=w4230:dbl[])
            n2364 = Divide(x=w4245, y=w4243) -> (x/y=w4229:dbl[])
            n2365 = Divide(x=w4244, y=w4243) -> (x/y=w4228:dbl[])
            n2366 = Divide(x=w4215, y=w4213) -> (x/y=w4214:dbl[])
            n2367 = Divide(x=w4212, y=w4210) -> (x/y=w4211:dbl[])
            n2368 = Build Array(w4231, w4230, w4246, w4229, w4228, w4243, w4214, w4213, w4211, w4210, w4207, w4206, w4205) -> (w4204:dbl[][])
            n2369 = Bundle("T1 Y", "T1 X", "T1 Sum", "T2 Y", "T2 X", "T2 Sum", "T1 FB X", "T1 FB Sum", "T2 FB X", "T2 FB Sum", "PSD Y", "PSD X", "PSD Y Sum") -> (w4232:T43)  [unwired: 1 out]
            n2370 = Cluster To Array(cluster=w4232) -> (array=w4241:string[])
          }
          frame "IR-QPD + PSD + FB-QPD XY positions" {
            w4306 = 4  # Channel pattern
            # "time average x2 the 3 psd signals (detection laser)"
            # "deinterlace 3 signals from qpds"
            n2371 = Decimate 1D Array(w4330) -> (w4329:i16[], w4328:i16[], w4307:i16[], w4327:i16[], w4273:i16[], w4319:i16[], w4318:i16[], w4295:i16[])
            n2372 = Decimate 1D Array "Feedback Sum"(w4307) -> (w4291:i16[], w4289:i16[])
            n2373 = Decimate 1D Array "QPD Y"(w4329) -> (w4326:i16[], w4309:i16[])
            n2374 = Decimate 1D Array "QPD X"(w4328) -> (w4325:i16[], w4323:i16[])
            n2375 = Decimate 1D Array "Feedback Y"(w4273) -> (w4272:i16[], w4271:i16[])
            n2376 = Decimate 1D Array "QPD Sum"(w4327) -> (w4324:i16[], w4322:i16[])
            n2377 = Decimate 1D Array "Feedback X"(w4295) -> (w4292:i16[], w4290:i16[])
            n2378 = call "downsample 1D array - double.vi"("Ave N"=2.0, "Array In"=w4319) -> ("Array Out"=w4294:dbl[])  [unwired: 1 out]
            n2379 = call "downsample 1D array - double.vi"("Ave N"=2.0, "Array In"=w4318) -> ("Array Out"=w4293:dbl[])  [unwired: 1 out]
            n2380 = Interleave 1D Arrays(w4326, w4325, w4324, w4309, w4323, w4322, w4272, w4292, w4291, w4271, w4290, w4289, w4294, w4293) -> (w4317:dbl[])
            n2381 = Divide(x=w4317, y=3276.7) -> (x/y=w4316:dbl[])
            n2382 = Decimate 1D Array(w4316) -> (w4315:dbl[], w4314:dbl[], w4313:dbl[], w4312:dbl[], w4311:dbl[], w4310:dbl[], w4268:dbl[], w4282:dbl[], w4266:dbl[], w4267:dbl[], w4280:dbl[], w4264:dbl[], w4278:dbl[], w4276:dbl[])
            n2383 = Negate(x=w4276) -> (-x=w4274:dbl[])
            n2384 = Divide(x=w4278, y=w4274) -> (x/y=w4277:dbl[])
            n2385 = Divide(x=w4267, y=w4264) -> (x/y=w4263:dbl[])
            n2386 = Divide(x=w4268, y=w4266) -> (x/y=w4265:dbl[])
            n2387 = Divide(x=w4315, y=w4313) -> (x/y=w4299:dbl[])
            n2388 = Divide(x=w4314, y=w4313) -> (x/y=w4298:dbl[])
            n2389 = Divide(x=w4312, y=w4310) -> (x/y=w4297:dbl[])
            n2390 = Divide(x=w4311, y=w4310) -> (x/y=w4296:dbl[])
            n2391 = Divide(x=w4282, y=w4266) -> (x/y=w4281:dbl[])
            n2392 = Divide(x=w4280, y=w4264) -> (x/y=w4279:dbl[])
            n2393 = Build Array(w4299, w4298, w4313, w4297, w4296, w4310, w4265, w4281, w4266, w4263, w4279, w4264, w4277, w4276) -> (w4275:dbl[][])
            n2394 = Bundle("T1 Y", "T1 X", "T1 Sum", "T2 Y", "T2 X", "T2 Sum", "T1 FB Y", "T1 FB X", "T1 FB Sum", "T2 FB Y", "T2 FB X", "T2 FB Sum", "PSD X", "PSD Y Sum") -> (w4262:T44)  [unwired: 1 out]
            n2395 = To Word Integer(number=w4317) -> (16bit integer=w4261:i16[])
            n2396 = Cluster To Array(cluster=w4262) -> (array=w4308:string[])
          }
        }
      }
    }
    "AI labels" <- w3336
    n2397 = local read "APD Integration Time (s)"() -> (w3309:dbl)
    n2398 = Array Size(array=w3351) -> (size(s)=w3396:i32)
    n2399 = call <vilib>:"Std Deviation and Variance.vi"("X"=w3298) -> ("standard deviation"=w3297:dbl)  [unwired: 1 in, 2 out]
    n2400 = Add Array Elements(numeric array=w3298) -> (sum=w3299:u32)
    n2401 = Add Array Elements(numeric array=w3351) -> (sum=w3406:u32)
    n2402 = call <vilib>:"Std Deviation and Variance.vi"("X"=w3351) -> ("standard deviation"=w3350:dbl)  [unwired: 1 in, 2 out]
    n2403 = Divide(x=w3297, y=w3141) -> (x/y=w3294:dbl)
    "Rate sigma (Hz) 2" <- w3294
    n2404 = Multiply(x=w3141, y=w3396) -> (x*y=w3143:dbl)
    "Int. Time (s)" <- w3143
    n2405 = Divide(x=w3299, y=w3143) -> (x/y=w3295:dbl)
    "APD 2 Rate (Hz)" <- w3295
    n2406 = Multiply(x="APD Disp. Scale", y=w3302) -> (x*y=w3311:waveform(dbl)[])
    n2407 = Divide(x=w3406, y=w3143) -> (x/y=w3348:dbl)
    "APD 1 Rate (Hz)" <- w3348
    n2408 = Divide(x=w3350, y=w3141) -> (x/y=w3349:dbl)
    "Rate sigma (Hz)" <- w3349
    n2409 = Divide(x=w3294, y=w3295) -> (x/y=→"Sigma/Mean 2":dbl)
    n2410 = Multiply(x="APD Disp. Downsample", y=w3309) -> (x*y=w3307:dbl)
    n2411 = Divide(x=w3349, y=w3348) -> (x/y=→"Sigma/Mean":dbl)
    n2412 = Divide(x=w3311, y=w3307) -> (x/y=w3133:waveform(dbl)[])
    n2413 = Index Array(array=w3133, index=0) -> (element=w3291:waveform(dbl))
    n2414 = Index Array(array=w3133, index=1) -> (element=w3289:waveform(dbl))
    n2415 = Index Array(array=w3133, index=2) -> (element=w3135:waveform(dbl))
    n2416 = Subtract(x=w3291, y="APD 1 Offset") -> (x-y=w3287:waveform(dbl))
    n2417 = Subtract(x=w3289, y="APD 2 Offset") -> (x-y=w3286:waveform(dbl))
    n2418 = Subtract(x=w3135, y="APD 3 Offset") -> (x-y=w3132:waveform(dbl))
    n2419 = Add Array Elements(numeric array=w3142) -> (sum=w3145:u32)
    n2420 = call <vilib>:"Std Deviation and Variance.vi"("X"=w3142) -> ("standard deviation"=w3144:dbl)  [unwired: 1 in, 2 out]
    n2421 = Build Array(w3287, w3286, w3132) -> (→"APD Chart":waveform(dbl)[])
    n2422 = Divide(x=w3145, y=w3143) -> (x/y=w3139:dbl)
    "APD 3 Rate (Hz)" <- w3139
    n2423 = Divide(x=w3144, y=w3141) -> (x/y=w3140:dbl)
    "Rate sigma (Hz) 3" <- w3140
    n2424 = Divide(x=w3140, y=w3139) -> (x/y=→"Sigma/Mean 3":dbl)
    n2425 = local read "Data Period (s)"() -> (w3194:dbl)
    n2426 = local read "BD 1 Frequency 2 (MHz)"() -> (w3227:dbl)
    n2427 = local read "BD 1 Frequency 1 (MHz)"() -> (w3228:dbl)
    n2428 = Decimate 1D Array(w3235) -> (w3259:i16[], w3258:i16[], w3256:i16[], w3255:i16[])  [unwired: 9 out]
    n2429 = Multiply(x=w3194, y="Trap Pos. Disp. Downsample") -> (x*y=w3192:dbl)
    n2430 = Divide(x=w3259, y=w3258) -> (x/y=w3260:dbl[])
    n2431 = Divide(x=w3256, y=w3255) -> (x/y=w3257:dbl[])
    n2432 = local read "AOM X Cal (nm/MHz)"() -> (w3225:dbl)
    n2433 = Split 1D Array(array=w3260, index="N El. to Ave.") -> (second subarray=w3263:dbl[])  [unwired: 1 out]
    n2434 = Split 1D Array(array=w3257, index="N El. to Ave.") -> (second subarray=w3262:dbl[])  [unwired: 1 out]
    n2435 = Multiply(x=w3194, y="Trap Disp. Downsample") -> (x*y=w3273:dbl)
    "Display Period (s)" <- w3273
    n2436 = for "Trap AI" {
      tunnel: [w4055] -> w3438 mode=indexing
      tunnel: w3271 -> [w4046]
      tunnel: "Trap Disp. Downsample" -> [w4053]
      tunnel: w3337 -> [w4051] mode=indexing
      tunnel: w3194 -> [w4050]
      tunnel: w3336 -> [w4049] mode=indexing
      tunnel: [w4048] -> w3306 mode=indexing
      tunnel: w3273 -> [w4047]
      workers-P: _ -> [_]
      n2437 = Bundle By Name("Y"=w4051, "dt"=w4050) -> (w4052:waveform(dbl))  [unwired: 1 out]
      n2438 = Set Waveform Attribute(5:w4049, 6:"NI_ChannelName" ("name"), 7:w4052) -> (3:w4048:waveform(dbl))  [unwired: 1 in, 2 out]
      n2439 = call "downsample 1D array - double.vi"("Ave N"=w4053, "Array In"=w4051) -> ("Array Out"=w4054:dbl[])  [unwired: 1 out]
      n2440 = Bundle By Name(cluster=w4048, "t0"=w4046, "Y"=w4054, "dt"=w4047) -> (w4055:waveform(dbl))
    }
    n2441 = Bundle("BD 1 Frequency 1 (MHz)"=w3228, "BD 1 Frequency 2 (MHz)"=w3227) -> (w3229:T45)  [unwired: 1 out]
    n2442 = call-poly <vilib>:"Mean.vi"("X"=w3262) -> ("mean"=w3250:dbl)  [unwired: 1 out]
    n2443 = call-poly <vilib>:"Mean.vi"("X"=w3263) -> ("mean"=w3251:dbl)  [unwired: 1 out]
    n2444 = Reciprocal(x=w3273) -> (1/x=→"Trap Disp. Freq. (Hz)":dbl)
    n2445 = Cluster To Array(cluster=w3229) -> (array=w3226:dbl[])
    n2446 = local read "Trap X AI1 (DMA)"() -> (w3261:T13)
    n2447 = local read "Data points/scans (MCL)"() -> (w3416:dbl)
    n2448 = To Fixed-Point(number=w3250) -> (fixed-point=w3248:fxp<+/-,16,1>)  [unwired: 1 in]
    n2449 = To Fixed-Point(number=w3251) -> (fixed-point=w3249:fxp<+/-,16,1>)  [unwired: 1 in]
    n2450 = Bundle("Trap 1 Pos.", "Trap 2 Pos.") -> (w3270:cluster{string, string})  [unwired: 1 out]
    n2451 = Bundle By Name(cluster=w3261, "Set 1"=w3249, "Set 2"=w3248) -> (→"Trap X AI1 (DMA)":T13)
    n2452 = Cluster To Array(cluster=w3270) -> (array=w3267:string[])
    n2453 = Unbundle(w3130) -> (w3131:u32[])  [unwired: 2 out]
    n2454 = Select(t=-1.0, s="Negate Y Axis", f=1.0) -> (s? t:f=w3211:dbl)
    n2455 = for "Trap Position" {
      tunnel: w3275 -> [w3646] mode=indexing
      tunnel: "Trap Pos. Disp. Downsample" -> [w3645]
      tunnel: w3192 -> [w3643]
      tunnel: w3271 -> [w3642]
      tunnel: w3267 -> [w3640] mode=indexing
      tunnel: [w3639] -> w3181 mode=indexing
      tunnel: w3226 -> [w3637] mode=indexing
      tunnel: w3225 -> [w3635]
      tunnel: w3211 -> [w3634]
      n2456 = call "downsample 1D array - double.vi"("Ave N"=w3645, "Array In"=w3646) -> ("Array Out"=w3644:dbl[])  [unwired: 1 out]
      n2457 = Subtract(x=w3644, y=w3637) -> (x-y=w3638:dbl[])
      n2458 = Multiply(x=w3635, y=w3638) -> (x*y=w3636:dbl[])
      n2459 = Multiply(x=w3634, y=w3636) -> (x*y=w3633:dbl[])
      n2460 = Bundle By Name("Y"=w3633, "dt"=w3643, "t0"=w3642) -> (w3641:waveform(dbl))  [unwired: 1 out]
      n2461 = Set Waveform Attribute(5:w3640, 6:"NI_ChannelName" ("name"), 7:w3641) -> (3:w3639:waveform(dbl))  [unwired: 1 in, 2 out]
    }
    n2462 = To Double Precision Float(number=w3131) -> (double precision float=w3334:dbl[])
    n2463 = local read "Display Period (s)"() -> (w3323:dbl)
    n2464 = Increment(x=w3416) -> (x+1=w3417:dbl)
    n2465 = Index Array(array=w3181, index=0) -> (element=w3185:waveform(dbl))
    n2466 = Index Array(array=w3181, index=1) -> (element=w3180:waveform(dbl))
    n2467 = feedback #7(w3417) -> (w3420:dbl)
    n2468 = Select(t=0, s=w3407, f=w3420) -> (s? t:f=w3413:dbl)
    n2469 = Array Size(array=w3334) -> (size(s)=w3419:i32)
    n2470 = Build Array (concatenate)(w3302, w3438) -> (w3304:waveform(dbl)[])
    "All Signals" <- w3304
    n2471 = Add(x=w3419, y=w3413) -> (x+y=w3414:dbl)
    n2472 = Unbundle By Name(w3185) -> ("Y"=w3186:dbl[])
    n2473 = Divide(x="Bead Sep. Int. Time (s)", y=w3323) -> (x/y=w3221:dbl)
    n2474 = Add(x=w3186, y="FB Trap Pos Offset") -> (x+y=w3184:dbl[])
    "T1 x pos data" <- w3184
    n2475 = Greater?(x=w3414, y=w3416) -> (0:w3415:bool)
    n2476 = feedback #8(w3184) -> (w3223:dbl[])
    n2477 = Build Array (concatenate)(w3184, w3223) -> (w3222:dbl[])
    n2478 = Bundle By Name(cluster=w3185, "Y"=w3184) -> (w3183:waveform(dbl))
    n2479 = Select(t=w3413, s=w3415, f=w3414) -> (s? t:f=w3412:dbl)
    n2480 = feedback-in #7(w3412) -> ()
    n2481 = local read "MCL Scanning"() -> (w3410:bool)
    n2482 = Bundle(w3183, w3180) -> (w3179:cluster{waveform(dbl), waveform(dbl)})  [unwired: 1 out]
    n2483 = Split 1D Array(array=w3222, index=w3221) -> (first subarray=w3215:dbl[])  [unwired: 1 out]
    n2484 = feedback-in #8(w3215) -> ()
    n2485 = Not(x=w3415) -> (.not. x?=w3409:bool)
    n2486 = Cluster To Array(cluster=w3179) -> (array=w3155:waveform(dbl)[])
    "Trap Positions" <- w3155
    n2487 = call-poly <vilib>:"Mean.vi"("X"=w3215) -> ("mean"=w3214:dbl)  [unwired: 1 out]
    "Mean T1 Position (nm)" <- w3214
    n2488 = Subtract(x=w3215, y=w3214) -> (x-y=w3220:dbl[])
    n2489 = Square(x=w3220) -> (x^2=w3219:dbl[])
    n2490 = And(x=w3409, y=w3410) -> (x .and. y?=w3411:bool)
    n2491 = call-poly <vilib>:"Mean.vi"("X"=w3219) -> ("mean"=w3218:dbl)  [unwired: 1 out]
    n2492 = Square Root(x=w3218) -> (sqrt(x)=w3217:dbl)
    n2493 = Or(x=w3411, y=w3407) -> (x .or. y?=w3408:bool)
    n2494 = Equal?(x="Tab Control 6", y=T35."High Res Display") -> (x = y?=w3340:bool)
    n2495 = Multiply(x=10.0, y=w3217) -> (x*y=→"Trap 1 Position RMS (A)":dbl)
    n2496 = case "For displaying the high resolution display (no downsampling)" shown="True" w3340 {
      tunnel: w3306 -> [_ w3666]
      frame False {
      }
      frame True {
        n2497 = Index Array(array=w3666, index="High Res. Display") -> (element=w3667:waveform(dbl))
        n2498 = call <vilib>:"Std Deviation and Variance.vi"("X"=w3667) -> ("mean"=w3674:dbl, "standard deviation"=w3679:dbl)  [unwired: 1 in, 1 out]
        "Mean Intensity" <- w3674
        "Sigma" <- w3679
        n2499 = Subtract(x=w3667, y=w3674) -> (x-y=w3673:waveform(dbl))
        n2500 = Select(t=w3673, s="Subtract mean", f=w3667) -> (s? t:f=→"1 Channel":waveform(dbl))
        n2501 = Divide(x=w3679, y=w3674) -> (x/y=→"Sigma/Mean":dbl)
        n2502 = feedback #9(1) -> (w3668:i32)
        n2503 = Greater Or Equal?(x=w3668, y="Slow mean N ave.") -> (x >= y?=w3681:bool)
        n2504 = Increment(x=w3668) -> (x+1=w3683:i32)
        n2505 = Select(t=1, s=w3681, f=w3683) -> (s? t:f=w3670:i32)
        n2506 = feedback-in #9(w3670) -> ()
        n2507 = feedback #10() -> (w3671:waveform(dbl))  [unwired: 1 out]
        n2508 = case shown="Default" w3668 {
          tunnel: [w3686 w3689] -> w3672
          tunnel: w3671 -> [w3688 _]
          tunnel: w3667 -> [w3687 w3689]
          frame Default {
            n2509 = call-poly <vilib>:"Append Waveforms.vi"("waveform B"=w3687, "waveform A"=w3688) -> ("waveform out"=w3686:waveform(dbl))  [unwired: 1 in, 8 out]
          }
          frame 1 {
          }
        }
        n2510 = feedback-in #10(w3672) -> ()
        n2511 = case shown="True" w3681 {
          tunnel: w3672 -> [_ w3685]
          frame False {
          }
          frame True {
            n2512 = call-poly <vilib>:"Mean.vi"("X"=w3685) -> ("mean"=→"Slow mean":dbl)  [unwired: 1 out]
          }
        }
      }
    }
    n2513 = case "For plotting results of scanning MCL (fluorescence and detection laser images)" shown="True" w3408 {
      tunnel: w3407 -> [_ w3796]
      tunnel: w3416 -> [_ _]
      tunnel: w3306 -> [_ w3923]
      tunnel: w3284 -> [_ w3831]
      tunnel: w3130 -> [_ w3802]
      frame False {
      }
      frame True {
        w3812 = u32 0 items=["Horizontal", "Vertical", "Central", "1st Diagonal", "2nd Diagonal"] ("Type of Symmetry")
        w3838 = u32 0 items=["Horizontal", "Vertical", "Central", "1st Diagonal", "2nd Diagonal"] ("Type of Symmetry")